vi "scalar history.vi"   [LabVIEW 2021, in "Ring Buffer Strict Accessor Unit Tests.lvlib"]
uses:
  Ring Buffer Strict Accessor Unit Tests.lvlib
  Source/SubVIs/Endianess.ctl
  8b0cacaa-d5f0-40e7-ae51-ada40b281162.vi
  0304e6f6-8717-49aa-9cc9-78c1b5e777a1.vi
  3d4bbf4c-866c-47c5-b54c-b4658948d3d5.vi
  b4a04a6b-2970-4d05-bd81-b6e8d31407a0.vi
  26c6a96e-aa3f-457a-b785-d9c13bcca88d.vi
  f1b10b57-3b7a-4a4f-b6d0-d258e8ac8c0b.vi
  d8623002-0ecd-4a15-9142-111da97f192e.vi
  1d5788e3-82fd-4730-bb71-cc7ffd3e5b8a.vi
  dea59858-e716-43e9-baf5-2617991b618f.vi
  8b0cacaa-d5f0-40e7-ae51-ada40b281162.vi/4c2a6c61-f100-483c-8a49-51e57025a24c.vi
  8b0cacaa-d5f0-40e7-ae51-ada40b281162.vi/e57bc314-87c7-4952-9bc8-929005dac297.vi
  <userlib>/bjustice/Ring Buffer for Time Series Data/API Poly.vi
  <userlib>/bjustice/Ring Buffer for Time Series Data/API/Write Array.vi
  0304e6f6-8717-49aa-9cc9-78c1b5e777a1.vi/f2df9050-0eef-46c6-aff6-3ce3a8893ea5.vi
  3d4bbf4c-866c-47c5-b54c-b4658948d3d5.vi/17d75e1a-130a-47e0-8f2c-6c7d90b8ca77.vi
  <userlib>/bjustice/Ring Buffer for Time Series Data/API/Read Full Rotated Buffer.vi
  Source/SubVIs/Search for time to keep.vi
  Source/SubVIs/Index ByteArray.vi
  3d4bbf4c-866c-47c5-b54c-b4658948d3d5.vi/19bdd28a-0674-4be3-87bb-ec701e431d75.vi
  Source/SubVIs/error if empty buffer.vi
  b4a04a6b-2970-4d05-bd81-b6e8d31407a0.vi/4c2a6c61-f100-483c-8a49-51e57025a24c.vi
  b4a04a6b-2970-4d05-bd81-b6e8d31407a0.vi/e57bc314-87c7-4952-9bc8-929005dac297.vi
  26c6a96e-aa3f-457a-b785-d9c13bcca88d.vi/f2df9050-0eef-46c6-aff6-3ce3a8893ea5.vi
  f1b10b57-3b7a-4a4f-b6d0-d258e8ac8c0b.vi/17d75e1a-130a-47e0-8f2c-6c7d90b8ca77.vi
  f1b10b57-3b7a-4a4f-b6d0-d258e8ac8c0b.vi/19bdd28a-0674-4be3-87bb-ec701e431d75.vi
  d8623002-0ecd-4a15-9142-111da97f192e.vi/4c2a6c61-f100-483c-8a49-51e57025a24c.vi
  d8623002-0ecd-4a15-9142-111da97f192e.vi/e57bc314-87c7-4952-9bc8-929005dac297.vi
  1d5788e3-82fd-4730-bb71-cc7ffd3e5b8a.vi/f2df9050-0eef-46c6-aff6-3ce3a8893ea5.vi
  dea59858-e716-43e9-baf5-2617991b618f.vi/17d75e1a-130a-47e0-8f2c-6c7d90b8ca77.vi
  dea59858-e716-43e9-baf5-2617991b618f.vi/19bdd28a-0674-4be3-87bb-ec701e431d75.vi
  <userlib>/bjustice/Ring Buffer for Time Series Data/SubVIs/Split Values Array.vi
  <userlib>/bjustice/Ring Buffer for Time Series Data/SubVIs/Replace Values Array Multiple Timestamps.vi
  0304e6f6-8717-49aa-9cc9-78c1b5e777a1.vi/f2df9050-0eef-46c6-aff6-3ce3a8893ea5.vi/63c583a5-c20f-4aba-9c90-661423dee4c4.vi
  0304e6f6-8717-49aa-9cc9-78c1b5e777a1.vi/f2df9050-0eef-46c6-aff6-3ce3a8893ea5.vi/52385341-3d9c-45d2-aff5-e082a4793eb1.vi
  0304e6f6-8717-49aa-9cc9-78c1b5e777a1.vi/f2df9050-0eef-46c6-aff6-3ce3a8893ea5.vi/37f29efa-f142-46b1-a185-f0098a95fbb6.vi
  0304e6f6-8717-49aa-9cc9-78c1b5e777a1.vi/f2df9050-0eef-46c6-aff6-3ce3a8893ea5.vi/84b3d231-9afe-4b6e-afae-e0be43a31e4e.vi
  0304e6f6-8717-49aa-9cc9-78c1b5e777a1.vi/f2df9050-0eef-46c6-aff6-3ce3a8893ea5.vi/c726271c-fc36-4bb7-8553-8945ec40c1cd.vi
  0304e6f6-8717-49aa-9cc9-78c1b5e777a1.vi/f2df9050-0eef-46c6-aff6-3ce3a8893ea5.vi/a7b1d944-dc88-46f5-9d3e-305d46bbe1f6.vi
  0304e6f6-8717-49aa-9cc9-78c1b5e777a1.vi/f2df9050-0eef-46c6-aff6-3ce3a8893ea5.vi/8abc4a6e-a1d2-4e85-879b-517e0ab55733.vi
  0304e6f6-8717-49aa-9cc9-78c1b5e777a1.vi/f2df9050-0eef-46c6-aff6-3ce3a8893ea5.vi/bd347357-b475-4a03-9ac5-3b85ef11aecc.vi
  0304e6f6-8717-49aa-9cc9-78c1b5e777a1.vi/f2df9050-0eef-46c6-aff6-3ce3a8893ea5.vi/391b36e9-a702-45e4-9499-3914f8833a58.vi
  0304e6f6-8717-49aa-9cc9-78c1b5e777a1.vi/f2df9050-0eef-46c6-aff6-3ce3a8893ea5.vi/44155b33-c915-49ce-9e44-a66693aa70dd.vi
  0304e6f6-8717-49aa-9cc9-78c1b5e777a1.vi/f2df9050-0eef-46c6-aff6-3ce3a8893ea5.vi/36977d53-dbe0-4dbc-b2ac-3dea4345b868.vi
  3d4bbf4c-866c-47c5-b54c-b4658948d3d5.vi/17d75e1a-130a-47e0-8f2c-6c7d90b8ca77.vi/bbb64351-fa28-4ac1-b583-44e271193ecd.vi
  <userlib>/bjustice/Ring Buffer for Time Series Data/SubVIs/Rotate Buffer.vi
  Source/SubVIs/Search for oldest time to keep.vi
  Source/SubVIs/Search for newest time to keep.vi
  Source/SubVIs/datatype byte size.vi
  Source/SubVIs/array sizes to number of points.vi
  3d4bbf4c-866c-47c5-b54c-b4658948d3d5.vi/19bdd28a-0674-4be3-87bb-ec701e431d75.vi/81c66277-30bd-484c-9c7c-9646f36721bb.vi
  3d4bbf4c-866c-47c5-b54c-b4658948d3d5.vi/19bdd28a-0674-4be3-87bb-ec701e431d75.vi/7ca10173-70f1-4bfb-9c4b-948090662032.vi
  3d4bbf4c-866c-47c5-b54c-b4658948d3d5.vi/19bdd28a-0674-4be3-87bb-ec701e431d75.vi/ea4aced9-3494-4b3f-b998-02af6afbdac4.vi
  3d4bbf4c-866c-47c5-b54c-b4658948d3d5.vi/19bdd28a-0674-4be3-87bb-ec701e431d75.vi/022c581c-5349-49df-98f9-5a038829ee63.vi
  3d4bbf4c-866c-47c5-b54c-b4658948d3d5.vi/19bdd28a-0674-4be3-87bb-ec701e431d75.vi/ed40bcc8-bbaa-4b61-9e1a-b4b75cf21b06.vi
  3d4bbf4c-866c-47c5-b54c-b4658948d3d5.vi/19bdd28a-0674-4be3-87bb-ec701e431d75.vi/f4b703c2-aaab-40a0-b3da-b0c22dc82d50.vi
  3d4bbf4c-866c-47c5-b54c-b4658948d3d5.vi/19bdd28a-0674-4be3-87bb-ec701e431d75.vi/1efa054f-b143-4d96-9f7e-584a7c6fa7fd.vi
  3d4bbf4c-866c-47c5-b54c-b4658948d3d5.vi/19bdd28a-0674-4be3-87bb-ec701e431d75.vi/b7c29f3f-256a-4401-af9d-aa15374df391.vi
  3d4bbf4c-866c-47c5-b54c-b4658948d3d5.vi/19bdd28a-0674-4be3-87bb-ec701e431d75.vi/2fb7b479-974d-4a18-8674-c4c8d9dc9a89.vi
  3d4bbf4c-866c-47c5-b54c-b4658948d3d5.vi/19bdd28a-0674-4be3-87bb-ec701e431d75.vi/faac7175-5814-4bb6-a961-a8db1f460653.vi
  3d4bbf4c-866c-47c5-b54c-b4658948d3d5.vi/19bdd28a-0674-4be3-87bb-ec701e431d75.vi/b6af2a6f-71a4-4cfe-837f-b196861458b0.vi
  26c6a96e-aa3f-457a-b785-d9c13bcca88d.vi/f2df9050-0eef-46c6-aff6-3ce3a8893ea5.vi/63c583a5-c20f-4aba-9c90-661423dee4c4.vi
  26c6a96e-aa3f-457a-b785-d9c13bcca88d.vi/f2df9050-0eef-46c6-aff6-3ce3a8893ea5.vi/52385341-3d9c-45d2-aff5-e082a4793eb1.vi
  26c6a96e-aa3f-457a-b785-d9c13bcca88d.vi/f2df9050-0eef-46c6-aff6-3ce3a8893ea5.vi/37f29efa-f142-46b1-a185-f0098a95fbb6.vi
  26c6a96e-aa3f-457a-b785-d9c13bcca88d.vi/f2df9050-0eef-46c6-aff6-3ce3a8893ea5.vi/84b3d231-9afe-4b6e-afae-e0be43a31e4e.vi
  26c6a96e-aa3f-457a-b785-d9c13bcca88d.vi/f2df9050-0eef-46c6-aff6-3ce3a8893ea5.vi/c726271c-fc36-4bb7-8553-8945ec40c1cd.vi
  26c6a96e-aa3f-457a-b785-d9c13bcca88d.vi/f2df9050-0eef-46c6-aff6-3ce3a8893ea5.vi/a7b1d944-dc88-46f5-9d3e-305d46bbe1f6.vi
  26c6a96e-aa3f-457a-b785-d9c13bcca88d.vi/f2df9050-0eef-46c6-aff6-3ce3a8893ea5.vi/8abc4a6e-a1d2-4e85-879b-517e0ab55733.vi
  26c6a96e-aa3f-457a-b785-d9c13bcca88d.vi/f2df9050-0eef-46c6-aff6-3ce3a8893ea5.vi/bd347357-b475-4a03-9ac5-3b85ef11aecc.vi
  26c6a96e-aa3f-457a-b785-d9c13bcca88d.vi/f2df9050-0eef-46c6-aff6-3ce3a8893ea5.vi/391b36e9-a702-45e4-9499-3914f8833a58.vi
  26c6a96e-aa3f-457a-b785-d9c13bcca88d.vi/f2df9050-0eef-46c6-aff6-3ce3a8893ea5.vi/44155b33-c915-49ce-9e44-a66693aa70dd.vi
  26c6a96e-aa3f-457a-b785-d9c13bcca88d.vi/f2df9050-0eef-46c6-aff6-3ce3a8893ea5.vi/36977d53-dbe0-4dbc-b2ac-3dea4345b868.vi
  f1b10b57-3b7a-4a4f-b6d0-d258e8ac8c0b.vi/17d75e1a-130a-47e0-8f2c-6c7d90b8ca77.vi/bbb64351-fa28-4ac1-b583-44e271193ecd.vi
  f1b10b57-3b7a-4a4f-b6d0-d258e8ac8c0b.vi/19bdd28a-0674-4be3-87bb-ec701e431d75.vi/81c66277-30bd-484c-9c7c-9646f36721bb.vi
  f1b10b57-3b7a-4a4f-b6d0-d258e8ac8c0b.vi/19bdd28a-0674-4be3-87bb-ec701e431d75.vi/7ca10173-70f1-4bfb-9c4b-948090662032.vi
  f1b10b57-3b7a-4a4f-b6d0-d258e8ac8c0b.vi/19bdd28a-0674-4be3-87bb-ec701e431d75.vi/ea4aced9-3494-4b3f-b998-02af6afbdac4.vi
  f1b10b57-3b7a-4a4f-b6d0-d258e8ac8c0b.vi/19bdd28a-0674-4be3-87bb-ec701e431d75.vi/022c581c-5349-49df-98f9-5a038829ee63.vi
  f1b10b57-3b7a-4a4f-b6d0-d258e8ac8c0b.vi/19bdd28a-0674-4be3-87bb-ec701e431d75.vi/ed40bcc8-bbaa-4b61-9e1a-b4b75cf21b06.vi
  f1b10b57-3b7a-4a4f-b6d0-d258e8ac8c0b.vi/19bdd28a-0674-4be3-87bb-ec701e431d75.vi/f4b703c2-aaab-40a0-b3da-b0c22dc82d50.vi
  f1b10b57-3b7a-4a4f-b6d0-d258e8ac8c0b.vi/19bdd28a-0674-4be3-87bb-ec701e431d75.vi/1efa054f-b143-4d96-9f7e-584a7c6fa7fd.vi
  f1b10b57-3b7a-4a4f-b6d0-d258e8ac8c0b.vi/19bdd28a-0674-4be3-87bb-ec701e431d75.vi/b7c29f3f-256a-4401-af9d-aa15374df391.vi
  f1b10b57-3b7a-4a4f-b6d0-d258e8ac8c0b.vi/19bdd28a-0674-4be3-87bb-ec701e431d75.vi/2fb7b479-974d-4a18-8674-c4c8d9dc9a89.vi
  f1b10b57-3b7a-4a4f-b6d0-d258e8ac8c0b.vi/19bdd28a-0674-4be3-87bb-ec701e431d75.vi/faac7175-5814-4bb6-a961-a8db1f460653.vi
  f1b10b57-3b7a-4a4f-b6d0-d258e8ac8c0b.vi/19bdd28a-0674-4be3-87bb-ec701e431d75.vi/b6af2a6f-71a4-4cfe-837f-b196861458b0.vi
  1d5788e3-82fd-4730-bb71-cc7ffd3e5b8a.vi/f2df9050-0eef-46c6-aff6-3ce3a8893ea5.vi/63c583a5-c20f-4aba-9c90-661423dee4c4.vi
  1d5788e3-82fd-4730-bb71-cc7ffd3e5b8a.vi/f2df9050-0eef-46c6-aff6-3ce3a8893ea5.vi/52385341-3d9c-45d2-aff5-e082a4793eb1.vi
  1d5788e3-82fd-4730-bb71-cc7ffd3e5b8a.vi/f2df9050-0eef-46c6-aff6-3ce3a8893ea5.vi/37f29efa-f142-46b1-a185-f0098a95fbb6.vi
  1d5788e3-82fd-4730-bb71-cc7ffd3e5b8a.vi/f2df9050-0eef-46c6-aff6-3ce3a8893ea5.vi/84b3d231-9afe-4b6e-afae-e0be43a31e4e.vi
  1d5788e3-82fd-4730-bb71-cc7ffd3e5b8a.vi/f2df9050-0eef-46c6-aff6-3ce3a8893ea5.vi/c726271c-fc36-4bb7-8553-8945ec40c1cd.vi
  1d5788e3-82fd-4730-bb71-cc7ffd3e5b8a.vi/f2df9050-0eef-46c6-aff6-3ce3a8893ea5.vi/a7b1d944-dc88-46f5-9d3e-305d46bbe1f6.vi
  1d5788e3-82fd-4730-bb71-cc7ffd3e5b8a.vi/f2df9050-0eef-46c6-aff6-3ce3a8893ea5.vi/8abc4a6e-a1d2-4e85-879b-517e0ab55733.vi
  1d5788e3-82fd-4730-bb71-cc7ffd3e5b8a.vi/f2df9050-0eef-46c6-aff6-3ce3a8893ea5.vi/bd347357-b475-4a03-9ac5-3b85ef11aecc.vi
  1d5788e3-82fd-4730-bb71-cc7ffd3e5b8a.vi/f2df9050-0eef-46c6-aff6-3ce3a8893ea5.vi/391b36e9-a702-45e4-9499-3914f8833a58.vi
  1d5788e3-82fd-4730-bb71-cc7ffd3e5b8a.vi/f2df9050-0eef-46c6-aff6-3ce3a8893ea5.vi/44155b33-c915-49ce-9e44-a66693aa70dd.vi
  1d5788e3-82fd-4730-bb71-cc7ffd3e5b8a.vi/f2df9050-0eef-46c6-aff6-3ce3a8893ea5.vi/36977d53-dbe0-4dbc-b2ac-3dea4345b868.vi
  dea59858-e716-43e9-baf5-2617991b618f.vi/17d75e1a-130a-47e0-8f2c-6c7d90b8ca77.vi/bbb64351-fa28-4ac1-b583-44e271193ecd.vi
  dea59858-e716-43e9-baf5-2617991b618f.vi/19bdd28a-0674-4be3-87bb-ec701e431d75.vi/81c66277-30bd-484c-9c7c-9646f36721bb.vi
  dea59858-e716-43e9-baf5-2617991b618f.vi/19bdd28a-0674-4be3-87bb-ec701e431d75.vi/7ca10173-70f1-4bfb-9c4b-948090662032.vi
  dea59858-e716-43e9-baf5-2617991b618f.vi/19bdd28a-0674-4be3-87bb-ec701e431d75.vi/ea4aced9-3494-4b3f-b998-02af6afbdac4.vi
  dea59858-e716-43e9-baf5-2617991b618f.vi/19bdd28a-0674-4be3-87bb-ec701e431d75.vi/022c581c-5349-49df-98f9-5a038829ee63.vi
  dea59858-e716-43e9-baf5-2617991b618f.vi/19bdd28a-0674-4be3-87bb-ec701e431d75.vi/ed40bcc8-bbaa-4b61-9e1a-b4b75cf21b06.vi
  dea59858-e716-43e9-baf5-2617991b618f.vi/19bdd28a-0674-4be3-87bb-ec701e431d75.vi/f4b703c2-aaab-40a0-b3da-b0c22dc82d50.vi
  dea59858-e716-43e9-baf5-2617991b618f.vi/19bdd28a-0674-4be3-87bb-ec701e431d75.vi/1efa054f-b143-4d96-9f7e-584a7c6fa7fd.vi
  dea59858-e716-43e9-baf5-2617991b618f.vi/19bdd28a-0674-4be3-87bb-ec701e431d75.vi/b7c29f3f-256a-4401-af9d-aa15374df391.vi
  dea59858-e716-43e9-baf5-2617991b618f.vi/19bdd28a-0674-4be3-87bb-ec701e431d75.vi/2fb7b479-974d-4a18-8674-c4c8d9dc9a89.vi
  dea59858-e716-43e9-baf5-2617991b618f.vi/19bdd28a-0674-4be3-87bb-ec701e431d75.vi/faac7175-5814-4bb6-a961-a8db1f460653.vi
  dea59858-e716-43e9-baf5-2617991b618f.vi/19bdd28a-0674-4be3-87bb-ec701e431d75.vi/b6af2a6f-71a4-4cfe-837f-b196861458b0.vi
  <userlib>/bjustice/Ring Buffer for Time Series Data/SubVIs/Enforce array size multiple timestamps.vi
  Source/API/New.vi
  <vilib>/Utility/error.llb/Error Cluster From Error Code.vi
  <vilib>/Utility/error.llb/Trim Whitespace.vi
  <vilib>/addons/_JKI Toolkits/Caraya/classes/Assert/Assert Not Error.vi
  <vilib>/addons/_JKI Toolkits/Caraya/classes/Assert/Assert True.vi
  <vilib>/addons/_JKI Toolkits/Caraya/classes/Assert/Assert Equal Value_Variant.vi
  Source/Ring Buffer Strict Accessor.lvlib
  <vilib>/addons/_JKI Toolkits/Caraya/classes/Assert/Assert.lvclass
  <vilib>/addons/_JKI Toolkits/Caraya/classes/Test/Test.lvclass
types:
  T1 = typedef "Ring Buffer Strict Accessor.lvlib/Endianess.ctl" = enum16{"big-endian", "little-endian"}
  T2 = typedef "Ring Buffer Strict Accessor.lvlib/RingBufferHandle.ctl" = cluster{"Ring buffer DVR":refnum<data-value>, "Data Type":T3, "Size(s)":i32[], "Endianess":T1, "Buffer Size (#timestamps) [init]":i32}
  T3 = typedef "Ring Buffer Strict Accessor.lvlib/DataType.ctl" = enum16{"uint8", "uint16", "uint32", "uint64", "int8", "int16", "int32", "int64", "float", "double", "extended"}
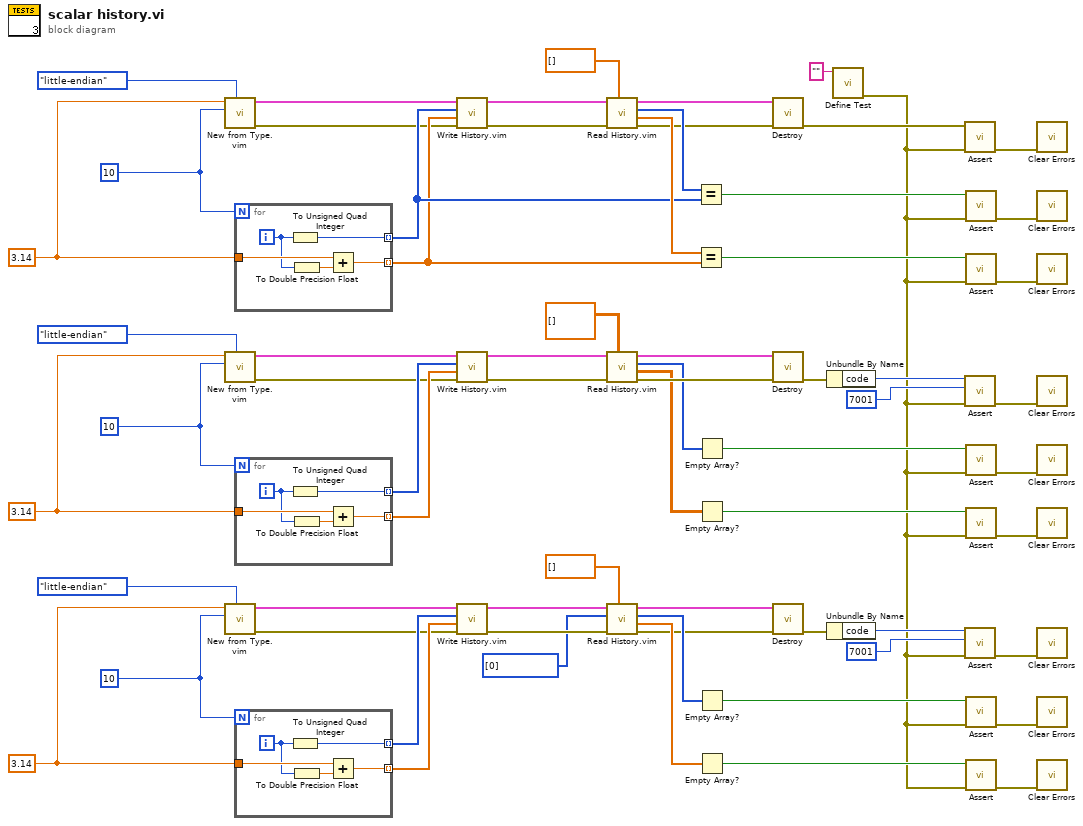
[diagram p0: block diagram]
diagram:
  w7 = 3.14 ("Numeric")
  w3 = 10 ("Buffer Size (#timestamps)")
  w8 = 3.14 ("Numeric")
  w4 = 10 ("Buffer Size (#timestamps)")
  w12 = 3.14 ("Numeric")
  w11 = 10 ("Buffer Size (#timestamps)")
  n1 = call "New from Type.vim"("Endianess"=Endianess."little-endian", "Buffer Size (#timestamps)"=w11, "LV type (array size cannot be empty)"=w12) -> ("error out"=w13:errorcluster, "Ring Buffer"=w14:T2)  [unwired: 7 in]
  n2 = call "New from Type.vim"("Endianess"=Endianess."little-endian", "Buffer Size (#timestamps)"=w4, "LV type (array size cannot be empty)"=w8) -> ("error out"=w1:errorcluster, "Ring Buffer"=w2:T2)  [unwired: 7 in]
  n3 = call "New from Type.vim"("Endianess"=Endianess."little-endian", "Buffer Size (#timestamps)"=w3, "LV type (array size cannot be empty)"=w7) -> ("error out"=w9:errorcluster, "Ring Buffer"=w10:T2)  [unwired: 7 in]
  n4 = for {
    N: w11 -> [_]
    tunnel: w12 -> [w72]
    tunnel: [w71] -> w52 mode=indexing
    tunnel: [w70] -> w53 mode=indexing
    i -> [w69]
    n5 = To Unsigned Quad Integer(1:w69) -> (0:w70:u64)
    n6 = To Double Precision Float(number=w69) -> (double precision float=w68:dbl)
    n7 = Add(x=w72, y=w68) -> (x+y=w71:dbl)
  }
  n8 = for {
    N: w4 -> [_]
    tunnel: w8 -> [w77]
    tunnel: [w76] -> w51 mode=indexing
    tunnel: [w75] -> w50 mode=indexing
    i -> [w74]
    n9 = To Unsigned Quad Integer(1:w74) -> (0:w75:u64)
    n10 = To Double Precision Float(number=w74) -> (double precision float=w73:dbl)
    n11 = Add(x=w77, y=w73) -> (x+y=w76:dbl)
  }
  n12 = for {
    N: w3 -> [_]
    tunnel: w7 -> [w82]
    tunnel: [w81] -> w18 mode=indexing
    tunnel: [w80] -> w19 mode=indexing
    i -> [w79]
    n13 = To Unsigned Quad Integer(1:w79) -> (0:w80:u64)
    n14 = To Double Precision Float(number=w79) -> (double precision float=w78:dbl)
    n15 = Add(x=w82, y=w78) -> (x+y=w81:dbl)
  }
  n16 = call "Write History.vim"("error in (no error)"=w13, "LV DataType"=w52, "Timestamps"=w53, "Ring Buffer"=w14) -> ("error out"=w62:errorcluster, "Ring Buffer"=w67:T2)  [unwired: 6 in]
  n17 = call "Write History.vim"("error in (no error)"=w1, "LV DataType"=w51, "Timestamps"=w50, "Ring Buffer"=w2) -> ("error out"=w45:errorcluster, "Ring Buffer"=w42:T2)  [unwired: 6 in]
  n18 = call "Write History.vim"("error in (no error)"=w9, "LV DataType"=w18, "Timestamps"=w19, "Ring Buffer"=w10) -> ("error out"=w24:errorcluster, "Ring Buffer"=w27:T2)  [unwired: 6 in]
  n19 = call "Read History.vim"("data type"=dbl[] [], "error in (no error)"=w62, "Ring Buffer"=w67) -> ("error out"=w61:errorcluster, "Values"=w63:dbl[], "Timestamps"=w64:u64[], "Ring Buffer"=w66:T2)  [unwired: 5 in]
  n20 = call "Read History.vim"("data type"=dbl[][] [], "error in (no error)"=w45, "Ring Buffer"=w42) -> ("error out"=w46:errorcluster, "Values"=w39:dbl[][], "Timestamps"=w41:u64[], "Ring Buffer"=w43:T2)  [unwired: 5 in]
  n21 = call "Read History.vim"("data type"=dbl[] [], "error in (no error)"=w24, "index"=i32[] [0], "Ring Buffer"=w27) -> ("error out"=w23:errorcluster, "Values"=w30:dbl[], "Timestamps"=w28:u64[], "Ring Buffer"=w26:T2)  [unwired: 4 in]
  n22 = Equal?(x=w64, y=w53) -> (x = y?=w60:bool)
  n23 = Equal?(x=w63, y=w52) -> (x = y?=w59:bool)
  n24 = Empty Array?(array=w41) -> (empty?=w40:bool)
  n25 = Empty Array?(array=w39) -> (empty?=w38:bool)
  n26 = Empty Array?(array=w28) -> (empty?=w29:bool)
  n27 = Empty Array?(array=w30) -> (empty?=w31:bool)
  n28 = call "Destroy.vi"("error in (no error)"=w61, "Ring Buffer"=w66) -> ("error out"=w58:errorcluster)  [unwired: 9 in]
  n29 = call "Destroy.vi"("error in (no error)"=w46, "Ring Buffer"=w43) -> ("error out"=w37:errorcluster)  [unwired: 9 in]
  n30 = call "Destroy.vi"("error in (no error)"=w23, "Ring Buffer"=w26) -> ("error out"=w32:errorcluster)  [unwired: 9 in]
  n31 = Unbundle By Name(w37) -> ("code"=w36:i32)
  n32 = Unbundle By Name(w32) -> ("code"=w33:i32)
  n33 = call <vilib>:"Define Test.vi"("Label (VI Title)"="") -> ("error out"=w17:errorcluster)  [unwired: 9 in, 1 out]
  n34 = call-poly <vilib>:"Assert.vi"("error in (no error)"=w17, "Not Error?"=w58) -> ("error out"=w56:errorcluster)  [unwired: 8 in, 1 out]
  n35 = call-poly <vilib>:"Assert.vi"("error in (no error)"=w17, "Y"=7001 ("code"), "X"=w36) -> ("error out"=w47:errorcluster)  [unwired: 7 in, 1 out]
  n36 = call-poly <vilib>:"Assert.vi"("error in (no error)"=w17, "Y"=7001 ("code"), "X"=w33) -> ("error out"=w22:errorcluster)  [unwired: 7 in, 1 out]
  n37 = call-poly <vilib>:"Assert.vi"("error in (no error)"=w17, "True?"=w60) -> ("error out"=w55:errorcluster)  [unwired: 8 in, 1 out]
  n38 = call-poly <vilib>:"Assert.vi"("error in (no error)"=w17, "True?"=w59) -> ("error out"=w54:errorcluster)  [unwired: 8 in, 1 out]
  n39 = call-poly <vilib>:"Assert.vi"("error in (no error)"=w17, "True?"=w40) -> ("error out"=w48:errorcluster)  [unwired: 8 in, 1 out]
  n40 = call-poly <vilib>:"Assert.vi"("error in (no error)"=w17, "True?"=w38) -> ("error out"=w49:errorcluster)  [unwired: 8 in, 1 out]
  n41 = call-poly <vilib>:"Assert.vi"("error in (no error)"=w17, "True?"=w29) -> ("error out"=w21:errorcluster)  [unwired: 8 in, 1 out]
  n42 = call-poly <vilib>:"Assert.vi"("error in (no error)"=w17, "True?"=w31) -> ("error out"=w20:errorcluster)  [unwired: 8 in, 1 out]
  n43 = call <vilib>:"Clear Errors.vi"("error in (no error)"=w56) -> ()  [unwired: 5 in, 2 out]
  n44 = call <vilib>:"Clear Errors.vi"("error in (no error)"=w55) -> ()  [unwired: 5 in, 2 out]
  n45 = call <vilib>:"Clear Errors.vi"("error in (no error)"=w54) -> ()  [unwired: 5 in, 2 out]
  n46 = call <vilib>:"Clear Errors.vi"("error in (no error)"=w47) -> ()  [unwired: 5 in, 2 out]
  n47 = call <vilib>:"Clear Errors.vi"("error in (no error)"=w48) -> ()  [unwired: 5 in, 2 out]
  n48 = call <vilib>:"Clear Errors.vi"("error in (no error)"=w49) -> ()  [unwired: 5 in, 2 out]
  n49 = call <vilib>:"Clear Errors.vi"("error in (no error)"=w22) -> ()  [unwired: 5 in, 2 out]
  n50 = call <vilib>:"Clear Errors.vi"("error in (no error)"=w21) -> ()  [unwired: 5 in, 2 out]
  n51 = call <vilib>:"Clear Errors.vi"("error in (no error)"=w20) -> ()  [unwired: 5 in, 2 out]
